vi "Main-Centering DNA Tether_ver2_YCC.vi"() -> ()   [LabVIEW 2014]
uses:
  Main-Calibration/WLC fitting/SubVI/WLC-Fitting Cluster.ctl
  Main-Stage-PI/(Global) Current handle and LaserPower_YCC.vi
panel:
  out "Initial Velocity Array":dbl[](array[numeric]) format="%.6f"
  out "XY Scan Range  (um)":dbl
  out "Y-Center (um)":dbl
  out "Final QPD Array":dbl[](array[numeric])
  out "Final Stage Array":dbl[](array[numeric])
  out "QPD raw":dbl[](array[numeric])
  out "Stage Array Shift (um)":dbl
  in  "Avg. time delay (ms)":dbl=18.0
  in  "Filter type":T1(ring)=enum."Moving-window avg"
  out "abs(min QPD)":dbl
  out "abs(max QPD)":dbl
  in  "WLC fit?":bool
  out "Guess-QPD-center (V)":dbl
  out "step size (nm)":dbl
  out "QPD height for tether (V)":dbl
  in  "Enum":enum16{"parity method", "max-min method"}(ring)=enum."max-min method"
  in  "Who's Data":enum16{"YCC", "PYW", "LCH", "YYH"}(ring)
  in  "File name add to the end \n(height)":string="h300"
  out "mean QPD":dbl
  out "Positon Start scan point (um)":dbl
  out "Filtered QPD data":dbl[](array[numeric])
  out "Filtered Stage Array":dbl[](array[numeric])
  in  "Save Data?":bool
  out "Running time":dbl
  in  "Move to new Center?":bool=TRUE
  in  "no record \nscan rate  (um/s)":dbl=4.0
  out "need time":dbl
  out "True rate?":bool
  out "Sample points want to record":dbl
  out "X-Center (um)":dbl
  out "Move to":dbl
  in  "Tab Control":enum32{"Filter", "Raw+Filter", "WLC fitting"}(tab)
  out "Filtered stage-QPD Graph":cluster{"X":dbl[], "Filtered X":dbl[]}[](graph)
  out "Raw+Filter stage-QPD Graph":cluster{"Raw Stage Array":dbl[], "data":dbl[]}[](graph)
  out "Force-Extension Graph":cluster{"Raw Stage Array":dbl[], "data":dbl[]}[](graph)=[{"Raw Stage Array"=[-1611.6314235823843, -1602.3016430258976, -1588.4786522996064, -1573.2964388258197, -1556.3301466356488, -1541.4110435671655, -1524.4367768488814, -1505.0139132361842, -1486.184264049311, -1465.390686222454, -1444.9186760893379, -1425.054597864122, -1407.7526998546773, -1383.9855217167728, -1366.3862277468922, -1341.1363077400674, -1318.6941624569106, -1298.2906950956003, -1280.2016041733752, -1258.5059747393327, -1235.9736542566782, -1215.2737671005605, -1199.2473796426264, -1180.6926593336984, -1153.6719049660312, -1129.673975630899, -1108.533770590797, -1095.159365510428, -1068.9153508024929, -1048.9404877814784, -1028.5738770161283, -1008.4601133264091, -989.3222931161713, -966.3299698496326, -952.8029095071677, -926.4251624080496, -905.1727087276051, -888.9266039247582, -871.4668686178561, -848.7098454653303, -829.1939795555795, -811.7698016661932, -786.73248831059, -778.9414508331474, -762.0791173090468, -735.9402483853389, -726.2112027122259, -704.5071495997886, -684.3453839331166, -672.2371298868957, -647.9555256125432, -640.3326407202567, -629.6538795429685, -599.534409109677, -588.0963932261604, -577.1908569978741, -557.1012225433526, 555.6808692720836, 561.5525700941523, 576.1793379824326, 595.4540102628207, 609.5824675269077, 624.6361193008602, 640.9197769689536, 645.5681831226498, 679.6248486905681, 688.635136681791, 717.0032859681016, 726.9899379100611, 742.9442503954276, 765.8557683094539, 778.28208522979, 800.4666905968845, 813.7520114546312, 830.2591825746449, 850.0742232956982, 870.1477733366708, 889.6341809139633, 908.3938889372967, 930.2836521832389, 950.7300322780416, 977.8692444214803, 995.7604138371446, 1015.8312183762064, 1031.0564471575012, 1051.1187179829433, 1073.2570497176625, 1098.2740679580784, 1112.7278103185172, 1140.111291858158, 1158.8160792718318, 1177.2323466369844, 1201.8537925594396, 1222.5367744769198, 1240.625525097813, 1264.895199366346, 1285.449839259901, 1306.3466956667282, 1331.0389643783267, 1350.3523900982357, 1372.0293895920338, 1388.8699677687448, 1411.002979343031, 1433.5118943928207, 1454.4062185877392, 1481.304272551801, 1495.6518477862373, 1518.1937856554546, 1537.7317787015818, 1558.006213152341, 1579.142775362856, 1594.1662092477923, 1611.9191979087364, 1628.2333800201554, 1642.7304545796378, 1654.255812633664, 1663.0381099881774], "data"=[-4.619998548066525, -4.005572471227063, -3.3022153618765437, -2.7281920516463165, -2.251916375207191, -1.9323475796116725, -1.648084951150685, -1.396765707668434, -1.206999706714476, -1.0417323648548718, -0.9123251872320108, -0.8103101789112829, -0.736039929604035, -0.6511836249370292, -0.5985064949095346, -0.534717329690212, -0.48730893184936463, -0.450254874400878, -0.42137850518764025, -0.39085941113044576, -0.3631395387512894, -0.3406618747537138, -0.32493938274320755, -0.3083285331926873, -0.28677050492614586, -0.2698476852707544, -0.256411703948687, -0.24853767154033546, -0.23432851352877093, -0.22449038345022293, -0.21522093151780564, -0.20673870931348826, -0.19922291956916927, -0.1908326848620167, -0.18619189402121106, -0.17770740971065163, -0.171362169424419, -0.16677756257647164, -0.16208576291019194, -0.1563056440274651, -0.15162461116918552, -0.14764213561743034, -0.1422167164682933, -0.1405949597728549, -0.13718574700139652, -0.1321552452670842, -0.13035633395516966, -0.1264762624450823, -0.12302581971205409, -0.12102009602349131, -0.1171378188556507, -0.11595549825016606, -0.11432701506799833, -0.10989886148305766, -0.10827722208398816, -0.10675997309163636, -0.10403529391971404, 0.0014215525813350213, 0.002142058764181755, 0.003963988927407812, 0.006426577280037239, 0.00827866978036177, 0.010298233618042503, 0.012539310394545533, 0.013190284409655757, 0.01812187301097326, 0.019477139201330304, 0.023894524496113248, 0.025507202784060157, 0.02815011931687425, 0.03209792199818037, 0.03431931808065901, 0.03843646869488121, 0.04100101474264746, 0.04429830208024721, 0.04843000033044491, 0.052824746265727585, 0.057310174172040526, 0.06185053494636866, 0.0674499944206425, 0.07300235161221688, 0.08090830061771818, 0.08649182788345293, 0.09314690619295572, 0.09849732698685089, 0.10598564201166509, 0.11488947033098094, 0.12586634014709913, 0.13270525334836164, 0.14679891536400946, 0.15739233266974456, 0.16869785172565394, 0.18536268530751815, 0.20094106353632185, 0.21593217967250228, 0.23837549826385873, 0.25982480970780203, 0.2843503318705872, 0.317557624121137, 0.3473640996901984, 0.3856835289813016, 0.41970134490074384, 0.4712917135077818, 0.5336660048722858, 0.6029002912940847, 0.7131388079707097, 0.7844698979331872, 0.9198311618029702, 1.0672739113470415, 1.2608325318436235, 1.5242464447722892, 1.7649642194242237, 2.1307514261955567, 2.577304860070708, 3.103501371496199, 3.6461682391663985, 4.161439407506152]}, {"Raw Stage Array"=[-1611.6314235823843, -1602.3016430258976, -1588.4786522996064, -1573.2964388258197, -1556.3301466356488, -1541.4110435671655, -1524.4367768488814, -1505.0139132361842, -1486.184264049311, -1465.390686222454, -1444.9186760893379, -1425.054597864122, -1407.7526998546773, -1383.9855217167728, -1366.3862277468922, -1341.1363077400674, -1318.6941624569106, -1298.2906950956003, -1280.2016041733752, -1258.5059747393327, -1235.9736542566782, -1215.2737671005605, -1199.2473796426264, -1180.6926593336984, -1153.6719049660312, -1129.673975630899, -1108.533770590797, -1095.159365510428, -1068.9153508024929, -1048.9404877814784, -1028.5738770161283, -1008.4601133264091, -989.3222931161713, -966.3299698496326, -952.8029095071677, -926.4251624080496, -905.1727087276051, -888.9266039247582, -871.4668686178561, -848.7098454653303, -829.1939795555795, -811.7698016661932, -786.73248831059, -778.9414508331474, -762.0791173090468, -735.9402483853389, -726.2112027122259, -704.5071495997886, -684.3453839331166, -672.2371298868957, -647.9555256125432, -640.3326407202567, -629.6538795429685, -599.534409109677, -588.0963932261604, -577.1908569978741, -557.1012225433526, 555.6808692720836, 561.5525700941523, 576.1793379824326, 595.4540102628207, 609.5824675269077, 624.6361193008602, 640.9197769689536, 645.5681831226498, 679.6248486905681, 688.635136681791, 717.0032859681016, 726.9899379100611, 742.9442503954276, 765.8557683094539, 778.28208522979, 800.4666905968845, 813.7520114546312, 830.2591825746449, 850.0742232956982, 870.1477733366708, 889.6341809139633, 908.3938889372967, 930.2836521832389, 950.7300322780416, 977.8692444214803, 995.7604138371446, 1015.8312183762064, 1031.0564471575012, 1051.1187179829433, 1073.2570497176625, 1098.2740679580784, 1112.7278103185172, 1140.111291858158, 1158.8160792718318, 1177.2323466369844, 1201.8537925594396, 1222.5367744769198, 1240.625525097813, 1264.895199366346, 1285.449839259901, 1306.3466956667282, 1331.0389643783267, 1350.3523900982357, 1372.0293895920338, 1388.8699677687448, 1411.002979343031, 1433.5118943928207, 1454.4062185877392, 1481.304272551801, 1495.6518477862373, 1518.1937856554546, 1537.7317787015818, 1558.006213152341, 1579.142775362856, 1594.1662092477923, 1611.9191979087364, 1628.2333800201554, 1642.7304545796378, 1654.255812633664, 1663.0381099881774], "data"=[-4.656331538320399, -3.8084461070653592, -3.251172830611154, -2.787798064672793, -2.439009327088495, -1.9845292157142729, -1.65733338730838, -1.4732662914013395, -1.2634433975625414, -1.1648949075948312, -1.0539931607666804, -0.9165062351140741, -0.6540993488901481, -0.7268848756065142, -0.4932293274115758, -0.6457442848259081, -0.6615575962267384, -0.5810582089855589, -0.39489607393824494, -0.38764894463971666, -0.42376233912729416, -0.37791867591725714, -0.12414777273946788, 0.004367063961370927, -0.24878261733566898, -0.3703208935074885, -0.36815455867967817, -0.03535573077930816, -0.26343884982060134, -0.2275034210196394, -0.2139931946368769, -0.1956833201696689, -0.14364079452257436, -0.2535157870308172, 0.007880708733146695, -0.24376154685691953, -0.29885304048712347, -0.1665727048823705, -0.091036125736684, -0.22007780957113945, -0.23417049276557486, -0.1791905181464599, -0.4066557736545147, -0.026580305473547193, 0.019196383871574855, -0.25636206574637155, 0.013207818276638136, -0.12398410358224288, -0.21748245028286128, -0.060907989218056784, -0.299489407974829, -0.026025274270545937, 0.13154967254791855, -0.29512616998505536, -0.1739558388273493, -0.05369818151475777, -0.2066291121905965, -0.109813013478337, 0.12159468417347535, 0.1250327011355979, 0.004721771985849636, 0.04189983388413213, 0.06302216229895827, 0.057378148283017176, 0.4301108955180409, -0.11623277722902314, 0.1340740893508399, -0.22020096354780538, 0.018927299014104802, 0.07948776311737933, -0.0852830595436472, 0.11285210067784957, -0.016269085487450298, 0.1755749016578684, 0.2651409290585137, 0.24092891436249364, 0.21332530441479663, 0.2143163871956805, 0.2502487054224633, 0.17034180551838773, 0.15221010200191465, -0.12520582329568222, -0.03375276838683196, -0.021958649843900845, 0.1963924194552362, 0.2231105358165979, 0.1669350796982022, -0.008141864970017005, 0.2763307424207767, 0.003508320966189304, 0.11449223907540171, 0.2464266597997362, 0.10339144654648232, 0.14246817318307858, 0.30740467156010304, 0.18934956533827474, 0.2491426665046238, 0.2976932601205266, 0.16781621869663907, 0.3007859347640948, 0.32381429959744373, 0.5927056856942676, 0.6024964201337047, 0.5964781647019127, 0.6768021743849892, 0.45041803132867636, 0.8796428750157154, 0.8858833543580209, 1.0563993985695193, 1.1927484557023376, 1.2865969248330489, 1.7258101103770704, 2.022804356007883, 2.411263881813612, 2.917286047950265, 3.615866720938015, 4.503208321440456]}]
  in  "Fitting Cluster":T2={"cr (um)"=0.0, "yr (V)"=0.0, "trap height(nm)"=0.0, "bead radius(nm)"=520.0, "Length offset"=0.0, "Upper Force(pN)"=0.0, "cr shift (nm)"=0.0, "yr shift (mV)"=0.0, "LaserPower (mW)"=0.0, "conversion factor (V/um)"=0.0, "Stiffness (pN/nm)"=0.0, "xDNA cut outside"=3000.0, "Lower Force(pN)"=5.0, "c for zbd"=0.0}
  in  "bead radius(nm)":dbl=515.0
  in  "trap height(nm)":dbl=300.0
  in  "Length offset":dbl=550.0
  in  "Force offset":dbl=5.0
  in  "initial parameters for marko":dbl[](array[numeric])=[40.0, 1800.0, 0.001, 0.001]
  out "best fit parameters\n(Lp,Lc,dL,dF)":dbl[](array[numeric])=[46.52503582812475, 1762.9522593141617, 28.337288191082056, -0.04759947195837781]
  out "r^2":dbl=0.9693121873029144
  in  "Avg points":i32=400
  out "total time to travel (s)":dbl
  out "Axis":i32
  in  "T=+ first\nF=- first":bool
  out "Real initial position (um)":dbl format="%0.5f"
  in  "Sampling rate (Hz)":dbl=32000.0 format="%0.2f"
  in  "scan rate  (um/s)":dbl=2.0 format="%.3f"
  in  "Scan Range  (um)":dbl=2.7999999999999985 format="%.3f"
  in  "X=T,Y=F":bool=TRUE
  # "range=2.6um for 5180 bp"
  # "3.6 um for fully coated 5180bp"
  # "0.54V for h=300 at 1000mV"
  # "3281bp : 1109.0 nm ~ 1115.5 nm (0.338 ~ 0.34)"
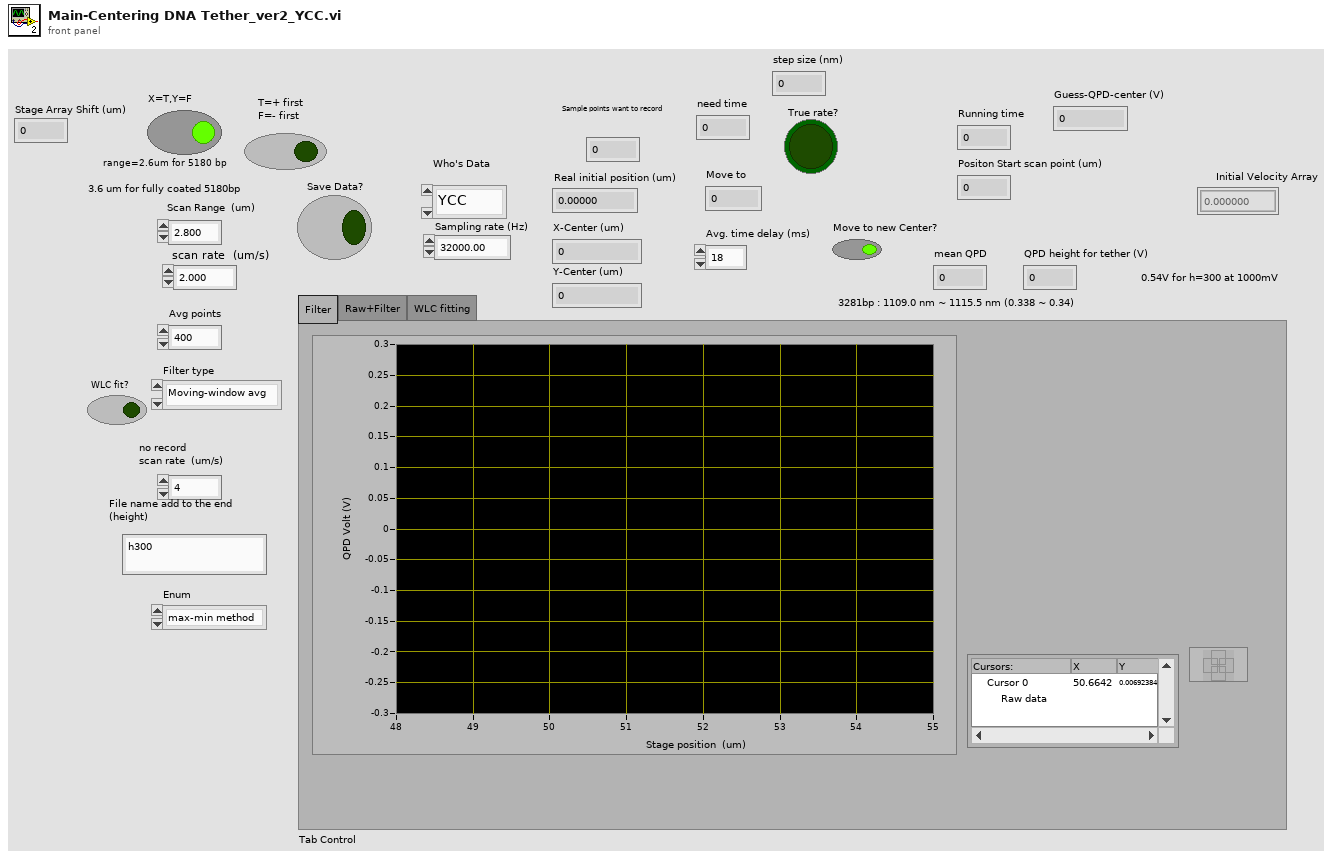
[diagram p1: front panel]
types:
  T1 = enum16{"Fixed-window avg", "Moving-window avg", "F+S-window avg", "S-G filter", "Fixed-window Median", "Moving-window Median "}
  T2 = typedef "WLC-Fitting Cluster.ctl" = cluster{"cr (um)":dbl, "yr (V)":dbl, "trap height(nm)":dbl, "bead radius(nm)":dbl, "Length offset":dbl, "Upper Force(pN)":dbl, "cr shift (nm)":dbl, "yr shift (mV)":dbl, "LaserPower (mW)":dbl, "conversion factor (V/um)":dbl, "Stiffness (pN/nm)":dbl, "xDNA cut outside":dbl, "Lower Force(pN)":dbl, "c for zbd":dbl}
  T3 = cluster{"Correct Unfolded Stage Array (um)":dbl[], "Filtered QPD data":dbl[]}
  T4 = cluster{"Raw Stage Array":dbl[], "Array":dbl[]}[]
  T5 = cluster{"Correct Unfolded Stage Array (um)":dbl[], "Filtered QPD data":dbl[]}[]
  T6 = cluster{"xDNA":dbl[], "best nonlinear fit for Force (pN)":dbl[]}
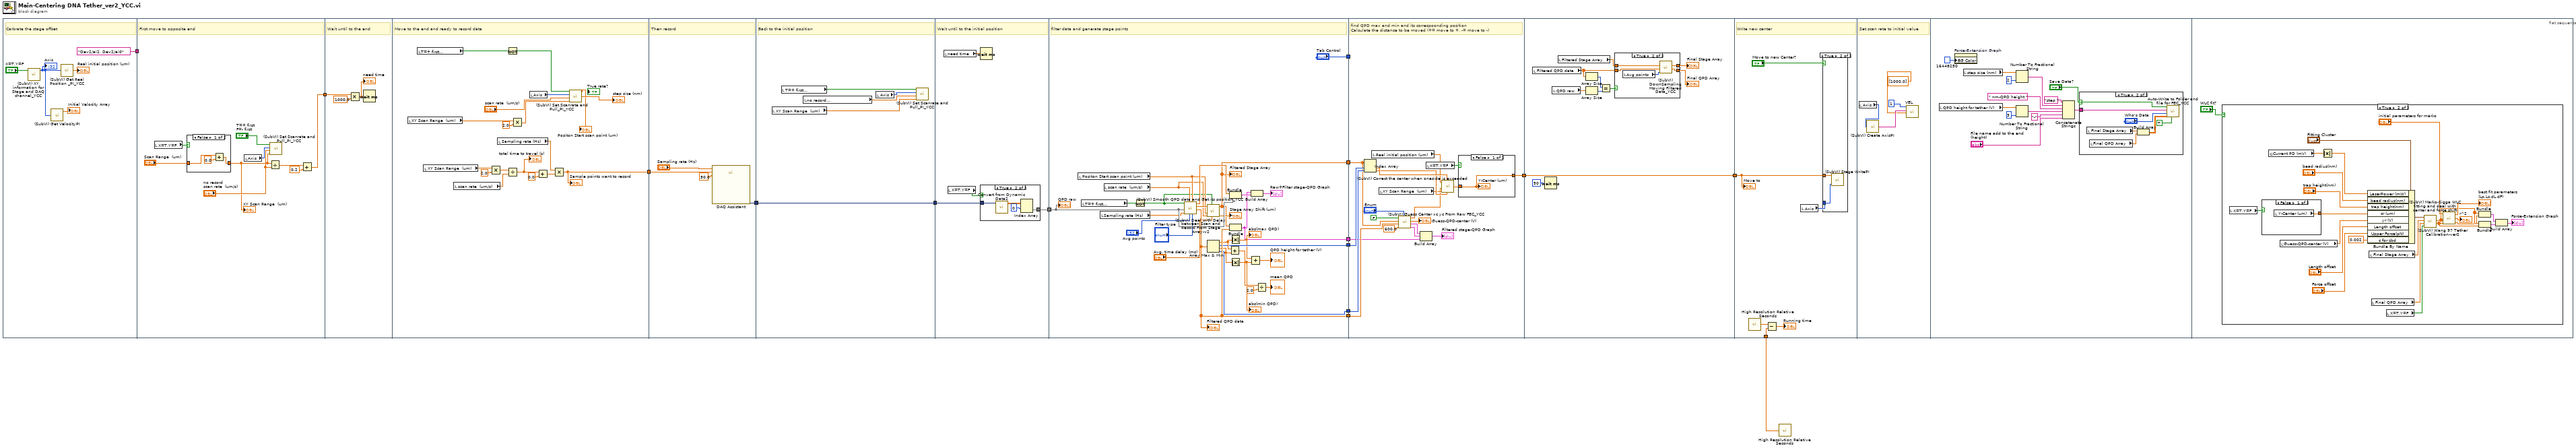
[diagram p0: block diagram]
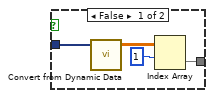
[diagram p3: hidden frame]
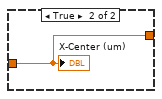
[diagram p4: hidden frame]
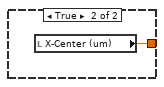
[diagram p9: hidden frame]
diagram:
  n1 = flat-sequence {
    tunnel: [tag "Dev2/ai2, Dev2/ai0" ("physical channels")] -> w15
    tunnel: [w26] -> w11
    tunnel: w15 -> [_]
    tunnel: w11 -> [w36]
    tunnel: [w43] -> w7
    tunnel: [w56] -> w10
    tunnel: w7 -> [w57]
    tunnel: w10 -> [w63]
    tunnel: [w63] -> w9
    tunnel: w9 -> [w66]
    tunnel: [w64] -> w8
    tunnel: w8 -> [w102]
    tunnel: [w96] -> w14
    tunnel: [w80] -> w13
    tunnel: ["Tab Control"] -> w12
    tunnel: [w89] -> w5
    tunnel: [w88] -> w4
    tunnel: [w77] -> w3
    tunnel: w14 -> [w121]
    tunnel: w13 -> [w110]
    tunnel: w12 -> [_]
    tunnel: w5 -> [w118]
    tunnel: w4 -> [w117]
    tunnel: w3 -> [w106]
    tunnel: [w104] -> w1
    tunnel: [w126] -> w2
    tunnel: w1 -> [w126]
    tunnel: w6 -> [w145]
    tunnel: w2 -> [w143]
    frame #0 {
      # "Carbrate the stage offset"
      n2 = call "(SubVI) XY information for Stage and DAQ channel_YCC.vi"("T=X\nF=Y"="X=T,Y=F") -> ("Axis"=w17:i32)  [unwired: 3 in, 1 out]
      "Axis" <- w17
      n3 = call "(SubVI) Get VelocityPI.vi"("axis"=w17) -> ("Velocity Array"=→"Initial Velocity Array":dbl[])  [unwired: 3 in, 1 out]
      n4 = call "(SubVI) Get Real Position _PI_YCC.vi"("Axis"=w17) -> ("Real Current Commanded position (um)"=→"Real initial position (um)":dbl)  [unwired: 4 in]
    }
    frame #1 {
      # "First move to opposite end"
      n5 = local read "X=T,Y=F"() -> (w22:bool)
      n6 = case shown="False" w22 {
        tunnel: [w30 w33] -> w23
        tunnel: "Scan Range  (um)" -> [w32 w33]
        frame False {
          n7 = Add(x=w32, y=0.0) -> (x+y=w30:dbl)
        }
        frame True {
        }
      }
      "XY Scan Range  (um)" <- w23
      n8 = local read "Axis"() -> (w29:i32)
      n9 = Divide(x=w23, y="no record \nscan rate  (um/s)") -> (x/y=w28:dbl)
      n10 = call "(SubVI) Set Scanrate and Pull_PI_YCC.vi"("toward+ ?\nT=+, F=-"="T=+ first\nF=- first", "axis"=w29, "scan rate  (um/s)"="no record \nscan rate  (um/s)", "range  (um)"=w23) -> ()  [unwired: 3 in, 2 out]
      n11 = Add(x=w28, y=0.2) -> (x+y=w26:dbl)
    }
    frame #2 {
      # "Wait until to the end"
      n12 = Multiply(x=w36, y=1000.0) -> (x*y=w34:dbl)
      "need time" <- w34
      n13 = Wait (ms)(milliseconds to wait=w34) -> ()  [unwired: 1 out]
    }
    frame #3 {
      # "Move to the end and ready to record data"
      n14 = local read "XY Scan Range  (um)"() -> (w38:dbl)
      n15 = local read "T=+ first\nF=- first"() -> (w41:bool)
      n16 = local read "XY Scan Range  (um)"() -> (w45:dbl)
      n17 = local read "scan rate  (um/s)"() -> (w44:dbl)
      n18 = Multiply(x=w45, y=2.0) -> (x*y=w47:dbl)
      n19 = local read "Sampling rate (Hz)"() -> (w40:dbl)
      n20 = Not(x=w41) -> (.not. x?=w51:bool)
      n21 = Divide(x=w47, y=w44) -> (x/y=w48:dbl)
      "total time to travel (s)" <- w48
      n22 = Multiply(x=w38, y=2.0) -> (x*y=w52:dbl)
      n23 = local read "Axis"() -> (w42:i32)
      n24 = Add(x=w48, y=0.0) -> (x+y=w49:dbl)
      n25 = Multiply(x=w40, y=w49) -> (x*y=w43:dbl)
      "Sample points want to record" <- w43
      n26 = call "(SubVI) Set Scanrate and Pull_PI_YCC.vi"("toward+ ?\nT=+, F=-"=w51, "axis"=w42, "scan rate  (um/s)"="scan rate  (um/s)", "range  (um)"=w52) -> ("Start From  (um)"=→"Positon Start scan point (um)":dbl, "Traveling time (s)"=→"step size (nm)":dbl)  [unwired: 3 in]
    }
    frame #4 {
      # "Then record"
      n27 = call "DAQ Assistant"("rate"="Sampling rate (Hz)", "number of samples"=w57, "timeout (s)"=50.0) -> ("data"=w56:dynamicdata)  [unwired: 13 in, 3 out]
    }
    frame #5 {
      # "Back to the initial position"
      n28 = local read "XY Scan Range  (um)"() -> (w59:dbl)
      n29 = local read "T=+ first\nF=- first"() -> (w60:bool)
      n30 = local read "no record \nscan rate  (um/s)"() -> (w62:dbl)
      n31 = local read "Axis"() -> (w61:i32)
      n32 = call "(SubVI) Set Scanrate and Pull_PI_YCC.vi"("toward+ ?\nT=+, F=-"=w60, "axis"=w61, "scan rate  (um/s)"=w62, "range  (um)"=w59) -> ()  [unwired: 3 in, 2 out]
    }
    frame #6 {
      # "Wait until to the initial position"
      n33 = local read "need time"() -> (w67:dbl)
      n34 = local read "X=T,Y=F"() -> (w65:bool)
      n35 = Wait (ms)(milliseconds to wait=w67) -> ()  [unwired: 1 out]
      n36 = case shown="True" w65 {
        tunnel: w66 -> [w70 w75]
        tunnel: [w69 w73] -> w64
        frame False {
          n37 = call "Convert from Dynamic Data"("Dynamic Data Type"=w70) -> ("Array"=w68:dbl[][])  [unwired: 3 in]
          n38 = Index Array(array=w68, index (row)=1) -> (element=w69:dbl[])  [unwired: 1 in]
        }
        frame True {
          n39 = call "Convert from Dynamic Data2"("Dynamic Data Type"=w75) -> ("Array"=w72:dbl[][])  [unwired: 3 in]
          n40 = Index Array(array=w72, index (row)=0) -> (element=w73:dbl[])  [unwired: 1 in]
        }
      }
    }
    frame #7 {
      # "filter data and generate stage points"
      n41 = local read "Positon Start scan point (um)"() -> (w79:dbl)
      n42 = local read "T=+ first\nF=- first"() -> (w83:bool)
      n43 = local read "Sampling rate (Hz)"() -> (w101:dbl)
      n44 = local read "scan rate  (um/s)"() -> (w78:dbl)
      n45 = Not(x=w83) -> (.not. x?=w76:bool)
      n46 = call "(SubVI) Smooth QPD data and Get its position_YCC.vi"("Filter type"="Filter type", "Initial position (um)"=w79, "Avg points"="Avg points", "scan rate  (um/s)"=w78, "Sampling rate (Hz)"=w101, "QPD data"=w102, "Direction\nT=+ \nF=-"=w76) -> ("Filtered QPD data"=w96:dbl[], "Filtered Stage Array"=w84:dbl[], "Raw Stage Array"=w99:dbl[])  [unwired: 2 in]
      "Filtered QPD data" <- w96
      n47 = call "(SubVI) Deal with Delay between Scan and Record From Stage Array-v2.vi"("Avg. time delay (ms)"="Avg. time delay (ms)", "Toward first ?\nT=+, F=-"=w76, "Record scan rate  (um/s)"=w78, "Real initial position (um)"=w79, "Unfolded Stage Array (um)"=w84) -> ("Stage Array Shift (nm)"=→"Stage Array Shift (um)":dbl, "Correct Unfolded Stage Array (um)"=w80:dbl[])  [unwired: 2 in, 1 out]
      "Filtered Stage Array" <- w80
      n48 = Array Max & Min(array=w96) -> (max value=w92:dbl, max index (indices)=w89:i32, min value=w91:dbl, min index (indices)=w88:i32)
      n49 = Add(x=w92, y=w91) -> (x+y=w95:dbl)
      n50 = Bundle("Raw Stage Array"=w99, "Array"=w102) -> (w98:cluster{"Raw Stage Array":dbl[], "Array":dbl[]})  [unwired: 1 in]
      n51 = Bundle("Correct Unfolded Stage Array (um)"=w80, "Filtered QPD data"=w96) -> (w77:T3)  [unwired: 1 in]
      n52 = Absolute Value(x=w92) -> (abs(x)=w87:dbl)
      "abs(max QPD)" <- w87
      n53 = Absolute Value(x=w91) -> (abs(x)=w86:dbl)
      "abs(min QPD)" <- w86
      n54 = Add(x=w87, y=w86) -> (x+y=→"QPD height for tether (V)":dbl)
      n55 = Build Array(w77, w98) -> (→"Raw+Filter stage-QPD Graph":T4)
      n56 = Divide(x=w95, y=2.0) -> (x/y=→"mean QPD":dbl)
      "QPD raw" <- w102
    }
    frame #8 {
      # "find QPD max and min and its correspoonding position\nCalculate the distance to be moved (+= move to +, -= move to -)"
      n57 = Index Array(array=w110, index #1=w118, index #2=w117) -> (element #1=w116:dbl, element #2=w115:dbl)
      n58 = local read "Real initial position (um)"() -> (w112:dbl)
      n59 = local read "XY Scan Range  (um)"() -> (w114:dbl)
      n60 = call "(SubVI) Guess Center xc yc From Raw FEC_YCC.vi"("Enum"="Enum", "avg range for QPD center (nm)"=600.0, "QPD array (V)"=w121, "Stage array(um)"=w110, "Read data?"=FALSE) -> ("Best Fit for min"=w108:cluster{"X":dbl[], "Best Polynomial Fit":dbl[]}, "Best Fit for max"=w109:cluster{"X":dbl[], "Best Polynomial Fit":dbl[]}, "Guess-QPD-center (V)"=→"Guess-QPD-center (V)":dbl, "Guess-stage-center(um)"=w113:dbl)  [unwired: 1 in]
      n61 = Build Array(w109, w108, w106) -> (→"Filtered stage-QPD Graph":T5)
      n62 = local read "X=T,Y=F"() -> (w105:bool)
      n63 = call "(SubVI) Correct the center when oneside is exceeded.vi"("initial position (um)"=w112, "maxQPD position (um)"=w116, "Guess center (um)"=w113, "minQPD position (um)"=w115, "range (um)"=w114) -> ("Correct center (um)"=w111:dbl)  [unwired: 3 in]
      n64 = case shown="False" w105 {
        tunnel: w111 -> [w124 w125]
        tunnel: [w124 w125] -> w104
        frame False {
          "Y-Center (um)" <- w124
        }
        frame True {
          "X-Center (um)" <- w125
        }
      }
    }
    frame #9 {
      n65 = local read "Filtered QPD data"() -> (w129:dbl[])
      n66 = Wait (ms)(milliseconds to wait=u32 50) -> ()  [unwired: 1 out]
      n67 = local read "QPD raw"() -> (w134:dbl[])
      n68 = local read "Filtered Stage Array"() -> (w130:dbl[])
      n69 = Array Size(array=w129) -> (size(s)=w133:i32)
      n70 = Array Size(array=w134) -> (size(s)=w132:i32)
      n71 = Equal?(x=w133, y=w132) -> (x = y?=w131:bool)
      n72 = case shown="True" w131 {
        tunnel: w130 -> [w137 w141]
        tunnel: w129 -> [w136 w140]
        tunnel: [w136 w139] -> w128
        tunnel: [w137 w138] -> w127
        frame False {
        }
        frame True {
          n73 = local read "Avg points"() -> (w142:i32)
          n74 = call "(SubVI) DownSampling Moving Filtered Data_YCC.vi"("data# reduce factor"=w142, "Moving Filtered QPD data"=w140, "Moving Filtered Stage data"=w141) -> ("DownSampling QPD"=w139:dbl[], "DownSampling Stage"=w138:dbl[])  [unwired: 3 in]
        }
      }
      "Final Stage Array" <- w127
      "Final QPD Array" <- w128
    }
    frame #10 {
      # "Write new center"
      n75 = call <vilib>:"High Resolution Relative Seconds.vi"() -> ("relative seconds"=w146:dbl)
      n76 = Subtract(x=w146, y=w145) -> (x-y=→"Running time":dbl)
      n77 = local read "Axis"() -> (w147:i32)
      n78 = case shown="True" "Move to new Center?" {
        tunnel: w143 -> [_ w150]
        tunnel: w147 -> [_ w149]
        frame False {
        }
        frame True {
          n79 = call "(SubVI) Stage WritePI.vi"("axis"=w149, "position"=w150) -> ()  [unwired: 4 in]
        }
      }
      "Move to" <- w143
    }
    frame #11 {
      # "Set scan rate to initial value"
      n80 = local read "Axis"() -> (w152:i32)
      n81 = call "(SubVI) Create AxisPI.vi"("axis"=w152) -> ("Axis String Array"=w153:string[])  [unwired: 2 in, 2 out]
      n82 = call "VEL.vi"("System no."=1, "Axes to set"=w153, "Velocity values"=dbl[] [1000.0]) -> ()  [unwired: 3 in, 14 out]
    }
    frame #12 {
      n83 = local read "QPD height for tether (V)"() -> (w160:dbl)
      n84 = property on="Force-Extension Graph" class="XYGraph (strict)"("BG Color"=u32 16448250) -> ()  [unwired: 2 in, 2 out]
      n85 = local read "step size (nm)"() -> (w166:dbl)
      n86 = Number To Fractional String(number=w166, precision (6)=i16 2) -> (F-format string=w162:string)  [unwired: 2 in]
      n87 = Number To Fractional String(number=w160, precision (6)=i16 3) -> (F-format string=w158:string)  [unwired: 2 in]
      n88 = Concatenate Strings("step " ("string"), w162, " nm-QPD height " ("string"), w158, "-" ("string"), "File name add to the end \n(height)") -> (w161:string)
      n89 = case shown="True" "Save Data?" {
        selector: "Save Data?" -> [_ w172]
        tunnel: w161 -> [_ w168]
        frame False {
        }
        frame True {
          n90 = local read "Final Stage Array"() -> (w174:dbl[])
          n91 = local read "Final QPD Array"() -> (w173:dbl[])
          n92 = Build Array(w174, w173) -> (w170:dbl[][])
          n93 = call "Auto-Write to Folder and file for FEC_YCC.vi"("Centering data?"=TRUE, "data to be saved"=w170, "Who's Data"="Who's Data", "File name add to the end \n(height)"=w168, "Save?"=w172) -> ()  [unwired: 3 in, 2 out]
        }
      }
    }
    frame #13 {
      n94 = case shown="True" "WLC fit?" {
        frame False {
        }
        frame True {
          n95 = local read "X=T,Y=F"() -> (w176:bool)
          n96 = case shown="False" w176 {
            tunnel: [w200 w201] -> w193
            frame False {
              n97 = local read "Y-Center (um)"() -> (w200:dbl)
            }
            frame True {
              n98 = local read "X-Center (um)"() -> (w201:dbl)
            }
          }
          n99 = global read "(Global) Current handle and LaserPower_YCC.vi" "Current PD (mV)"() -> (w183:dbl)
          n100 = local read "Guess-QPD-center (V)"() -> (w192:dbl)
          n101 = Absolute Value(x=w183) -> (abs(x)=w182:dbl)
          n102 = Bundle By Name(cluster="Fitting Cluster", "LaserPower (mW)"=w182, "bead radius(nm)"="bead radius(nm)", "trap height(nm)"="trap height(nm)", "cr (um)"=w193, "yr (V)"=w192, "Length offset"="Length offset", "Upper Force(pN)"="Force offset", "c for zbd"=0.002) -> (w196:T2)
          n103 = local read "Final Stage Array"() -> (w199:dbl[])
          n104 = local read "Final QPD Array"() -> (w198:dbl[])
          n105 = local read "X=T,Y=F"() -> (w181:bool)
          n106 = call "(SubVI) Wang 97 Tether Calibration-ver2.vi"("X=T\nY=F"=w181, "QPD signal"=w198, "Stage Position"=w199, "Fitting Cluster"=w196) -> ("Force"=w179:dbl[], "xDNA"=w187:dbl[])  [unwired: 1 in, 1 out]
          n107 = call "(SubVI) Marko-Sigga WLC fitting and deal with center and force shift.vi"("Force (pN)"=w179, "Extension (nm)"=w187, "initial parameters for marko"="initial parameters for marko") -> ("best nonlinear fit for Force (pN)"=w180:dbl[], "r^2"=→"r^2":dbl, "best fit parameters\n(Lp,Lc,dL,dF)"=→"best fit parameters\n(Lp,Lc,dL,dF)":dbl[])  [unwired: 1 in]
          n108 = Bundle("xDNA"=w187, "best nonlinear fit for Force (pN)"=w180) -> (w186:T6)  [unwired: 1 in]
          n109 = Bundle("xDNA"=w187, "Force"=w179) -> (w185:cluster{"xDNA":dbl[], "Force":dbl[]})  [unwired: 1 in]
          n110 = Build Array(w186, w185) -> (→"Force-Extension Graph":cluster{"xDNA":dbl[], "Force":dbl[]}[])
        }
      }
    }
  }
  n111 = call <vilib>:"High Resolution Relative Seconds.vi"() -> ("relative seconds"=w6:dbl)
